vi "UHR-Fleezers Control (host) - Avogadro v2.vi"() -> ()   [LabVIEW 2014] (continued)
              tunnel: w5202 -> [_ w5212]
              frame False {
              }
              frame True {
                n3617 = xnode "Read/Write Control"("FPGA VI Reference In"=w5213, "error in"=w5212, "FPGA Trap Trig"=TRUE) -> ()  [unwired: 2 out]
              }
            }
            n3618 = case shown="True" w5204 {
              frame False {
              }
              frame True {
                w5215 = FALSE ("Value (Signaling)")
                n3619 = local write "Triggered"(w5215) -> ()
                n3620 = local write "Waiting"(TRUE ("Waiting")) -> ()
                n3621 = property on="Green Laser ON" class="Bool (strict)"("Val(Sgnl)"=w5215) -> ()  [unwired: 2 in, 2 out]
              }
            }
          }
          frame "Do nothing" {
          }
          frame "Initialize", Default {
            n3622 = Increment(x=w5226) -> (x+1=w5230:i32)
            n3623 = Select(t=1, s=w5219, f=w5230) -> (s? t:f=w5220:i32)
            n3624 = feedback #23(w5228) -> (w5234:dbl[])
            n3625 = Build Array (concatenate)(w5228, w5234) -> (w5227:dbl[])
            n3626 = Greater Or Equal?(x=w5220, y="Wait to get offset (n)") -> (x >= y?=w5223:bool)
            n3627 = Select(t=w5228, s=w5219, f=w5227) -> (s? t:f=w5229:dbl[])
            n3628 = feedback-in #23(w5229) -> ()
            n3629 = call-poly <vilib>:"Mean.vi"("X"=w5229) -> ("mean"=w5224:dbl)  [unwired: 1 out]
            n3630 = local write "Mean T1 Position\nto compare (nm)"(w5224) -> ()
            n3631 = case shown="True" w5219 {
              tunnel: w5222 -> [_ w5240]
              tunnel: w5221 -> [_ w5239]
              frame False {
              }
              frame True {
                w5236 = FALSE ("FPGA Trap Trig")
                n3632 = xnode "Read/Write Control"("FPGA VI Reference In"=w5240, "error in"=w5239, "FPGA Trap Trig"=w5236) -> ("FPGA VI Reference Out"=w5238:T40, "error out"=w5237:errorcluster)
                n3633 = xnode "Read/Write Control"("FPGA VI Reference In"=w5238, "error in"=w5237, "TTrig?"=w5236) -> ()  [unwired: 2 out]
              }
            }
            n3634 = Select(t="Wait for trigger", s=w5223, f="Initialize") -> (s? t:f=w5231:string)
            n3635 = case shown="True" w5223 {
              tunnel: w5224 -> [_ w5243]
              tunnel: w5222 -> [_ w5252]
              tunnel: w5221 -> [_ w5251]
              frame False {
                n3636 = local write "Waiting"(FALSE ("Waiting")) -> ()
                "Initializing" <- TRUE ("Initializing")
              }
              frame True {
                n3637 = local read "Threshold (nm)"() -> (w5255:dbl)
                n3638 = local read "AOM X Cal (nm/MHz)"() -> (w5254:dbl)
                n3639 = Add(x=w5243, y=w5255) -> (x+y=w5256:dbl)
                n3640 = Divide(x=w5256, y=w5254) -> (x/y=w5253:dbl)
                n3641 = call "IR AOM freq to word.vi"("Frequency In (MHz)"=w5253) -> ("Frequency Word Out (double)"=w5250:dbl)
                n3642 = local write "Initializing"(FALSE ("Initializing")) -> ()
                n3643 = local write "Waiting"(TRUE ("Waiting")) -> ()
                n3644 = To Quad Integer(1:w5250) -> (0:w5249:i64)
                n3645 = xnode "Read/Write Control"("FPGA VI Reference In"=w5252, "error in"=w5251, "FPGA TTrig Thresh"=w5249) -> ("FPGA VI Reference Out"=w5246:T40, "error out"=w5245:errorcluster)
                n3646 = xnode "Read/Write Control"("FPGA VI Reference In"=w5246, "error in"=w5245, "FPGA Trap Trig"=TRUE) -> ()  [unwired: 2 out]
              }
            }
          }
        }
      }
    }
    n3647 = feedback-in #21(w4778) -> ()
    n3648 = feedback-in #22(w4775) -> ()
    n3649 = xnode ("Read/Write Control")("FPGA VI Reference In"=w4570, "error in"=w4837) -> ("FPGA VI Reference Out"=w4567:T40, "error out"=w4763:errorcluster, "AI2 Y Sum Set 1"=w4879:i16, "AI2 Y Sum Set 2"=w4878:i16, "AI1 X Set 1"=w4794:fxp<+/-,16,1>, "AI1 X Set 2"=w4793:fxp<+/-,16,1>, "Trap Pos FB Int Signal"=→"Trap Pos FB Int Signal":fxp<+/-,24,9>, "Trap Pos FB Int-Norm Signal"=→"Trap Pos FB Int-Norm Signal":fxp<+/-,16,1>, "Trap Pos FB Action"=w4787:i64, "Scanning"=→"AOD Scanning":bool, "Scan I"=→"AOD Scan I":u64, "Scanning MCL"=w4881:bool, "Scan I (MCL)"=→"MCL Scan I":u64, "Green FB Sum"=w4844:i16, "Trap Pos FB Action"=w4761:i64, "TTrig Fin Thresh"=w4757:i64, "Red FB Intensity"=w4749:i16, "Blue Intensity"=w4744:i16, "BD1 Frequency Out 1"=w4709:u64)
    "MCL Scanning" <- w4881
    "Trap Pos FB Action" <- w4787
    n3650 = Divide(x=w4749, y=3276.7) -> (x/y=w4748:dbl)
    "Red laser intensity (V)" <- w4748
    n3651 = Divide(x=w4744, y=3276.7) -> (x/y=w4743:dbl)
    "Blue laser intensity (V)" <- w4743
    n3652 = Divide(x=w4844, y=3276.7) -> (x/y=w4747:dbl)
    "Green laser intensity (V)" <- w4747
    n3653 = local read "FB Trig Integrate"() -> (w4755:u32)
    n3654 = Divide(x=w4761, y=w4755) -> (x/y=w4754:dbl)
    "TTrig Sig (Int)" <- w4754
    n3655 = Bundle(w4747, w4748, w4743) -> (→"Fluorescence laser intensities plot":cluster{dbl, dbl, dbl})  [unwired: 1 in]
    n3656 = Divide(x=w4757, y=w4755) -> (x/y=w4752:dbl)
    "TTrig Fin Thresh (Int)" <- w4752
    n3657 = local read "AOM X Cal (nm/MHz)"() -> (w4760:dbl)
    n3658 = local read "AI2 (V)"() -> (w4880:cluster{"Set 1":dbl, "Set 2":dbl})
    n3659 = Bundle By Name(cluster=w4880, "Set 1"=w4879, "Set 2"=w4878) -> (w4711:cluster{"Set 1":dbl, "Set 2":dbl})
    n3660 = Divide(x=w4787, y=327.67) -> (x/y=→"Action (%)":dbl)
    n3661 = case shown="True" "Semi Passive Mode" {
      tunnel: w4617 -> [_ w5028]
      frame False {
      }
      frame True {
        n3662 = local read "Target Force (pN)"() -> (w5026:dbl)
        n3663 = Less?(x="Jump Force (pN)", y=w5026) -> (x < y?=w5024:bool)
        n3664 = case shown="False" w5024 {
          tunnel: "Jump Force (pN)" -> [w5034 w5037]
          tunnel: w5028 -> [w5033 w5036]
          tunnel: [w5032 w5035] -> w5027
          frame False {
            n3665 = Less?(x=w5034, y=w5033) -> (x < y?=w5032:bool)
          }
          frame True {
            n3666 = Greater?(x=w5037, y=w5036) -> (0:w5035:bool)
          }
        }
        n3667 = case shown="False" w5027 {
          frame False {
            n3668 = local read "Trap Pos. FB ON"() -> (w5029:bool)
            n3669 = case shown="False" w5029 {
              frame False {
              }
              frame True {
                n3670 = property on="Trap Pos. FB ON" class="Bool (strict)"("Val(Sgnl)"=FALSE) -> ()  [unwired: 2 in, 2 out]
              }
            }
          }
          frame True {
            n3671 = property on="Trap Pos. FB ON" class="Bool (strict)"("Val(Sgnl)"=TRUE) -> ()  [unwired: 2 in, 2 out]
          }
        }
      }
    }
    n3672 = local read "Trap X (AI1)"() -> (w4807:T19)
    n3673 = call "IR AOM word double to freq.vi"("Frequency Word In (double)"=w4752) -> ("Frequency Out (MHz)"=w4751:dbl)
    n3674 = call "IR AOM word double to freq.vi"("Frequency Word In (double)"=w4754) -> ("Frequency Out (MHz)"=w4753:dbl)
    n3675 = Divide(x=w4711, y=3276.7) -> (x/y=w4876:cluster{"Set 1":dbl, "Set 2":dbl})
    n3676 = Multiply(x=w4753, y=w4760) -> (x*y=w4759:dbl)
    "TTrig Sig (nm)" <- w4759
    n3677 = Multiply(x=w4751, y=w4760) -> (x*y=w4758:dbl)
    "TTrig Fin Thresh (nm)" <- w4758
    n3678 = local write "AI2 (V)"(w4876) -> ()
    n3679 = Bundle(cluster=w4807, "Trap 1"=w4794, "Trap 2"=w4793) -> (→"Trap X (AI1)":T19)
    n3680 = local read "Trap Pos. FB ON"() -> (w4702:bool)
    n3681 = local read "Dynamic Force FB (ronen)"() -> (w4703:bool)
    n3682 = Bundle(w4759, w4758) -> (→"TTrig":cluster{dbl, dbl})  [unwired: 1 in]
    n3683 = Compound Arithmetic op=AND(w4703, "Real time Offset file correction for setpoint", w4702) -> (w4704:bool)
    n3684 = case shown="True" w4704 {
      tunnel: w4709 -> [_ _]
      tunnel: w4640 -> [_ w5056]
      tunnel: w4567 -> [_ w5039]
      frame False {
      }
      frame True {
        # "Changed by Ronen - real time update of set point\naccording to offset file"
        n3685 = local read "T1 calibration"() -> (w5051:T12)
        n3686 = local read "Offset file step size"() -> (w5058:dbl)
        n3687 = local read "Setpoint offset\ncorrection values"() -> (w5055:dbl[])
        n3688 = Multiply(x="Target Force (pN)", y=2.0) -> (x*y=w5052:dbl)
        n3689 = local read "Negate Diff?"() -> (w5040:bool)
        n3690 = Unbundle By Name(w5051) -> ("alpha_x (nm/V)"=w5050:dbl, "kappa_x (pN/nm)"=w5049:dbl)
        n3691 = Divide(x=w5056, y=w5058) -> (x/y=w5059:dbl)
        n3692 = To Long Integer(number=w5059) -> (32bit integer=w5057:i32)
        n3693 = Index Array(array=w5055, index=w5057) -> (element=w5042:dbl)
        n3694 = Multiply(x=w5050, y=w5049) -> (x*y=w5048:dbl)
        n3695 = Select(t=1, s=w5040, f=-1) -> (s? t:f=w5043:i32)
        n3696 = Divide(x=w5052, y=w5048) -> (x/y=w5047:dbl)
        n3697 = Multiply(x=w5043, y=w5042) -> (x*y=w5041:dbl)
        n3698 = Add(x=w5047, y=w5041) -> (x+y=w5046:dbl)
        n3699 = To Fixed-Point(number=w5046) -> (fixed-point=w5038:fxp<+/-,16,1>)  [unwired: 1 in]
        "Actual Setpoint" <- w5038
        n3700 = xnode "Read/Write Control"("FPGA VI Reference In"=w5039, "Trap Pos. FB SP"=w5038) -> ()  [unwired: 1 in, 2 out]
      }
    }
    n3701 = local read "All FB On/Off"() -> (w4710:bool)
    n3702 = case shown="True" w4710 {
      tunnel: w4567 -> [_ w5083]
      frame False {
      }
      frame True {
        n3703 = local read "X RF Amplitude Limits (%)"() -> (w5082:T26)
        n3704 = xnode "Read/Write Control"("FPGA VI Reference In"=w5083) -> ("BD1 amplitude 1 out"=w5074:u16, "BD1 amplitude 2 out"=w5066:u16)  [unwired: 1 in, 2 out]
        n3705 = Unbundle By Name(w5082) -> ("Maximum"=w5065:dbl)
        n3706 = Scale By Power Of 2(n=i16 12, x=ext 1.0) -> (x*2^n=w5078:ext)
        n3707 = Scale By Power Of 2(n=i16 12, x=ext 1.0) -> (x*2^n=w5070:ext)
        n3708 = Subtract(x=w5078, y=ext 1.0) -> (x-y=w5080:ext)
        n3709 = Subtract(x=w5070, y=ext 1.0) -> (x-y=w5068:ext)
        n3710 = Multiply(x=w5074, y=ext 100.0) -> (x*y=w5081:ext)
        n3711 = Multiply(x=w5066, y=ext 100.0) -> (x*y=w5067:ext)
        n3712 = Divide(x=w5081, y=w5080) -> (x/y=w5061:ext)
        "T1 feedback amplitude" <- w5061
        n3713 = Divide(x=w5067, y=w5068) -> (x/y=w5060:ext)
        "T2 feedback amplitude" <- w5060
        n3714 = Greater?(x=w5060, y=w5065) -> (0:w5063:bool)
        n3715 = Greater?(x=w5061, y=w5065) -> (0:w5064:bool)
        n3716 = Or(x=w5064, y=w5063) -> (x .or. y?=w5062:bool)
        n3717 = case shown="True" w5062 {
          frame False {
          }
          frame True {
            n3718 = property on="All FB On/Off" class="Bool (strict)"("Val(Sgnl)"=FALSE) -> ()  [unwired: 2 in, 2 out]
          }
        }
      }
    }
    n3719 = flat-sequence "To save data" {
      tunnel: [w5800] -> w4899
      tunnel: [w5801] -> w4898
      tunnel: w4861 -> [w5794]
      tunnel: w4583 -> [w5798]
      tunnel: ["Save Calibration"] -> w4873
      tunnel: w4692 -> [w5797]
      tunnel: [w5790] -> w4870
      tunnel: [w5787] -> w4869
      tunnel: [w5784] -> w4868
      tunnel: w4860 -> [w5786]
      tunnel: w4648 -> [w5780]
      tunnel: [w5780] -> w4831
      tunnel: ["Start Saving"] -> w4816
      tunnel: [w5775] -> w4783
      tunnel: [w5774] -> w4782
      tunnel: [w5771] -> w4715
      tunnel: [w5767] -> w4708
      tunnel: w4899 -> [w6134]
      tunnel: w4898 -> [w6133]
      tunnel: w4693 -> [w6132]
      tunnel: w4873 -> [w6131]
      tunnel: w4870 -> [w6129]
      tunnel: w4869 -> [w6128]
      tunnel: w4868 -> [w6127]
      tunnel: w4687 -> [w6126]
      tunnel: w4691 -> [w6125]
      tunnel: w4831 -> [w6124]
      tunnel: w4816 -> [w6123]
      tunnel: w4571 -> [w6122]
      tunnel: w4742 -> [w6121]
      tunnel: w4783 -> [w6120]
      tunnel: w4782 -> [w6119]
      tunnel: w4644 -> [w6118]
      tunnel: w4653 -> [w6117]
      tunnel: w4690 -> [w6116]
      tunnel: w4715 -> [w6115]
      tunnel: w4708 -> [w6114]
      frame #0 {
        # "Changed by Ronen - we don't have a database so we disabled this"
        n3720 = Or(x="Save N Sets", y="Start Saving") -> (x .or. y?=w5781:bool)
        n3721 = To Double Precision Float(number=w5797) -> (double precision float=w5791:dbl)
        n3722 = Build Array(w5781, "Save Calibration", w5794, w5786, "Flow Cal") -> (w5796:bool[])
        n3723 = Compound Arithmetic op=OR("Save Calibration", w5794, w5781, w5786, "Flow Cal") -> (w5799:bool)
        n3724 = Boolean Array To Number(Boolean array=w5796) -> (number=w5793:u32)
        n3725 = feedback #24(FALSE ("Save APD Data\nwith Trap Data")) -> (w5776:bool)
        n3726 = feedback #25(refnum<k0> refnum) -> (w5802:refnum<file>)
        n3727 = feedback #26(FALSE ("Save APD Data\nwith Trap Data")) -> (w5785:bool)
        n3728 = feedback #27(0) -> (w5804:i32)
        n3729 = feedback #28() -> (w5792:u32)  [unwired: 1 out]
        n3730 = feedback #29(refnum<k0> refnum) -> (w5772:refnum<file>)
        n3731 = feedback #30(refnum<k0> refnum) -> (w5778:refnum<file>)
        n3732 = feedback #31(refnum<k0> refnum) -> (w5768:refnum<file>)
        n3733 = feedback #32(refnum<k0> refnum) -> (w5788:refnum<file>)
        n3734 = case shown="True" w5799 {
          tunnel: [w5813 1] -> w5800
          tunnel: w5804 -> [w5815 _]
          tunnel: [w5814 w5847] -> w5801
          tunnel: w5802 -> [w5814 _]
          tunnel: w5798 -> [_ w5865]
          tunnel: w5791 -> [_ w5863]
          tunnel: w5793 -> [_ w5866]
          tunnel: [w5812 w5846] -> w5790
          tunnel: w5792 -> [w5812 _]
          tunnel: [w5811 w5844] -> w5787
          tunnel: w5788 -> [w5811 _]
          tunnel: [w5810 w5843] -> w5784
          tunnel: w5785 -> [w5810 _]
          tunnel: "Start Saving" -> [_ w5841]
          tunnel: w5780 -> [_ w5840]
          tunnel: [w5809 w5833] -> w5774
          tunnel: w5778 -> [w5809 _]
          tunnel: [w5808 w5832] -> w5775
          tunnel: w5776 -> [w5808 _]
          tunnel: [w5807 w5818] -> w5771
          tunnel: w5772 -> [w5807 _]
          tunnel: [w5806 w5816] -> w5767
          tunnel: w5768 -> [w5806 _]
          frame False {
            n3735 = Increment(x=w5815) -> (x+1=w5813:i32)
          }
          frame True {
            w5817 = FALSE ("Start Saving")
            w5842 = 10.0  # File Version
            w5849 = FALSE ("prepend array or string size? (T)")
            w5848 = T53."big-endian, network order" ("byte order (0:big-endian, network order)")
            # "RG added position values of traps in the saved\nfile for AOD rasters and time series."
            # "Ronen Changed the create file - changed data folder to c:\\Data"
            # "Save trap position\ndata"
            n3736 = Array Size(array=w5840) -> (size(s)=w5839:i32)
            n3737 = To Double Precision Float(number=w5839) -> (double precision float=w5838:dbl)
            n3738 = local read "BD 1 Frequency 1 (MHz)"() -> (w5862:dbl)
            n3739 = local read "BD 2 Frequency 1 (MHz)"() -> (w5861:dbl)
            n3740 = local read "BD 1 Frequency 2 (MHz)"() -> (w5860:dbl)
            n3741 = local read "BD 2 Frequency 2 (MHz)"() -> (w5859:dbl)
            n3742 = local read "BD 1 Frequency 3 (MHz)"() -> (w5858:dbl)
            n3743 = local read "BD 2 Frequency 3 (MHz)"() -> (w5857:dbl)
            n3744 = local write "Flow Cal"(w5817) -> ()
            n3745 = local write "Save Calibration"(w5817) -> ()
            n3746 = local write "Start Saving"(w5817) -> ()
            n3747 = Build Array("Save APD Data\nwith Trap Data", "Save Trap Pos. Data") -> (w5835:bool[])
            n3748 = Boolean Array To Number(Boolean array=w5835) -> (number=w5834:u32)
            n3749 = Build Array(w5862, w5861, w5860, w5859, w5858, w5857) -> (w5856:dbl[])
            n3750 = case shown="1, Default" w5866 {
              tunnel: w5865 -> [w5972 w5999 w6031 w6069 w6106]
              tunnel: w5838 -> [w5977 w6006 w6051 w6088 w6111]
              tunnel: w5863 -> [w5976 w6005 w6050 w6087 w6110]
              tunnel: [w5973 w6001 w6042 w6079 w6107] -> w5854
              tunnel: [w5964 "Cal sets to save" w6032 w6070 w6093] -> w5846
              tunnel: w5856 -> [w5974 w6002 w6044 w6081 w6108]
              tunnel: "Save APD Data\nwith Trap Data" -> [w5971 w5988 w6029 w6067 w6105]
              tunnel: [w5971 w5986 w6029 w6067 w6105] -> w5843
              tunnel: w5842 -> [w5967 w5995 w6027 w6065 w6101]
              tunnel: w5841 -> [w5966 _ _ _ _]
              tunnel: [w5957 w5994 w6026 w6055 w6100] -> w5832
              tunnel: "Save Trap Pos. Data" -> [w5957 w5993 w6026 w6055 w6100]
              tunnel: w5834 -> [w5956 w5992 w6025 w6054 w6099]
              frame 1, Default {
                # "timeseries"
                n3751 = case shown="True" "Profile" {
                  tunnel: [w5980 w5984] -> w5961
                  tunnel: [w5980 w5983] -> w5960
                  tunnel: [w5980 w5982] -> w5959
                  tunnel: [w5980 w5981] -> w5958
                  frame False {
                    w5980 = 0.0 ("f")
                  }
                  frame True {
                    n3752 = local read "Current Position"() -> (w5985:cluster{dbl, dbl, dbl})
                    n3753 = local read "Y change (mm)"() -> (w5981:dbl)
                    n3754 = Unbundle(w5985) -> (w5984:dbl, w5983:dbl, w5982:dbl)
                  }
                }
                n3755 = local read "Save ave N"() -> (w5979:dbl)
                n3756 = local read "AOM X Cal (nm/MHz)"() -> (w5955:dbl)
                n3757 = local read "Piezo Trap X cal (nm/V)"() -> (w5954:dbl)
                n3758 = local read "Piezo Trap Y cal (nm/V)"() -> (w5953:dbl)
                n3759 = local read "Piezo trap x\noffset (V)"() -> (w5952:dbl)
                n3760 = local read "Piezo trap y\noffset (V)"() -> (w5951:dbl)
                n3761 = To Double Precision Float(number=w5956) -> (double precision float=w5970:dbl)
                n3762 = Multiply(x=w5979, y=w5972) -> (x*y=w5978:dbl)
                n3763 = Build Array(w5967, w5972, w5978, w5977, w5976, 0.0 ("f")) -> (w5975:dbl[])
                n3764 = Build Array(w5970, w5961, w5960, w5959, w5958) -> (w5968:dbl[])
                n3765 = Build Array(w5955, w5954, w5953, w5952, w5951) -> (w5950:dbl[])
                n3766 = Select(t=u32 4000000000, s=w5966, f="N sets to save") -> (s? t:f=w5964:u32)
                n3767 = Build Array (concatenate)(w5975, w5974, w5968, w5950) -> (w5973:dbl[])
              }
              frame 2 {
                w5997 = 0.0 ("f")
                w5987 = FALSE ("Save APD Data\nwith Trap Data")
                # "For diagnostics save trap position\ndata during cal"
                # "calibration"
                n3768 = Boolean To (0,1)(Boolean=w5987) -> (0, 1=w5991:i16)
                n3769 = Select(t=w5988, s="Save trap pos with cal", f=w5987) -> (s? t:f=w5986:bool)
                n3770 = Select(t=w5993, s="Save trap pos with cal", f=w5987) -> (s? t:f=w5994:bool)
                n3771 = Select(t=w5992, s="Save trap pos with cal", f=w5991) -> (s? t:f=w5990:u32)
                n3772 = To Double Precision Float(number=w5990) -> (double precision float=w5998:dbl)
                n3773 = Build Array(w5995, w5999, w5999, w6006, w6005, 1.0 ("t")) -> (w6003:dbl[])
                n3774 = Build Array(w5998, w5997, w5997, w5997, w5997) -> (w5996:dbl[])
                n3775 = Build Array (concatenate)(w6003, w6002, w5996) -> (w6001:dbl[])
                "Calibrating Trap..." <- TRUE ("Calibrating...")
              }
              frame 4 {
                # "scan dir (x/y = 0/1)"
                # "cycles/step"
                # "n scans (f/b)"
                # "steps"
                # "freq. range"
                # "AOD raster scan"
                n3776 = local read "MCL offset scanning range (V)"() -> (w6022:T4)
                n3777 = local read "Multiple-MCL offset?"() -> (w6017:bool)
                n3778 = local read "Piezo Trap Y cal (nm/V)"() -> (w6008:dbl)
                n3779 = local read "AOM X Cal (nm/MHz)"() -> (w6010:dbl)
                n3780 = local read "Piezo Trap X cal (nm/V)"() -> (w6011:dbl)
                n3781 = local read "Piezo trap x\noffset (V)"() -> (w6012:dbl)
                n3782 = local read "Piezo trap y\noffset (V)"() -> (w6013:dbl)
                n3783 = local read "Number of F/B Scans (AOD)"() -> (w6036:u16)
                n3784 = Boolean To (0,1)(Boolean="Offset raster?") -> (0, 1=w6015:i16)
                n3785 = call "Make Trap3 position array.vi"("MCL offset scanning range (V)"=w6022) -> ("X Data points"=w6021:u64, "Y data points"=w6020:u64)  [unwired: 3 out]
                n3786 = Boolean To (0,1)(Boolean=w6017) -> (0, 1=w6024:i16)
                n3787 = local read "Cycles/step (AOD)"() -> (w6038:u64)
                n3788 = local read "Scan Range (MHz)"() -> (w6041:dbl)
                n3789 = local read "Scan steps (AOD)"() -> (w6040:u64)
                n3790 = local read "Scan BD"() -> (w6048:bool)
                n3791 = To Double Precision Float(number=w6024) -> (double precision float=w6023:dbl)
                n3792 = local read "Save ave N"() -> (w6053:dbl)
                n3793 = To Double Precision Float(number=w6020) -> (double precision float=w6018:dbl)
                n3794 = Build Array(w6010, w6011, w6008, w6012, w6013) -> (w6009:dbl[])
                n3795 = To Double Precision Float(number=w6021) -> (double precision float=w6019:dbl)
                n3796 = Boolean To (0,1)(Boolean=w6048) -> (0, 1=w6047:i16)
                n3797 = To Double Precision Float(number=w6015) -> (double precision float=w6014:dbl)
                n3798 = To Double Precision Float(number=w6036) -> (double precision float=w6035:dbl)
                n3799 = To Double Precision Float(number=w6040) -> (double precision float=w6039:dbl)
                n3800 = To Double Precision Float(number=w6038) -> (double precision float=w6037:dbl)
                n3801 = To Double Precision Float(number=w6047) -> (double precision float=w6046:dbl)
                n3802 = Multiply(x=w6053, y=w6031) -> (x*y=w6052:dbl)
                n3803 = To Double Precision Float(number=w6025) -> (double precision float=w6030:dbl)
                n3804 = local read "N sets should be saved"() -> (w6033:dbl)
                n3805 = Build Array(w6030, w6023, w6019, w6018, w6014) -> (w6028:dbl[])
                n3806 = Build Array(w6046, w6041, w6039, w6037, w6035) -> (w6043:dbl[])
                n3807 = Build Array(w6027, w6031, w6052, w6051, w6050, 2.0 ("t")) -> (w6045:dbl[])
                n3808 = Build Array (concatenate)(w6045, w6044, w6028, w6043, w6009) -> (w6042:dbl[])
                n3809 = Round Toward +Infinity(x=w6033) -> (ceil(x): smallest int >= x=w6034:dbl)
                n3810 = To Unsigned Long Integer(number=w6034) -> (unsigned 32bit integer=w6032:u32)
              }
              frame 8 {
                w6062 = 0.0 ("f")
                # "MCL raster scan"
                n3811 = local read "Number of scans (MCL)"() -> (w6057:u64)
                n3812 = local read "2D or 1D Scan"() -> (w6059:bool)
                n3813 = local read "Scan lines (y)"() -> (w6056:u64)
                n3814 = local read "Scan Range (V)\n(of steps)"() -> (w6078:dbl)
                n3815 = local read "Fast Scan Dir"() -> (w6085:bool)
                n3816 = local read "Cycles/step (MCL)"() -> (w6075:u64)
                n3817 = local read "Scan steps (MCL)"() -> (w6077:u64)
                n3818 = Select(t=w6056, s=w6059, f=w6057) -> (s? t:f=w6058:u64)
                n3819 = Boolean To (0,1)(Boolean=w6059) -> (0, 1=w6061:i16)
                n3820 = local read "Save ave N"() -> (w6090:dbl)
                n3821 = local read "Initial X"() -> (w6064:dbl)
                n3822 = local read "Initial Y"() -> (w6063:dbl)
                n3823 = To Double Precision Float(number=w6061) -> (double precision float=w6060:dbl)
                n3824 = Boolean To (0,1)(Boolean=w6085) -> (0, 1=w6084:i16)
                n3825 = To Double Precision Float(number=w6058) -> (double precision float=w6073:dbl)
                n3826 = To Double Precision Float(number=w6077) -> (double precision float=w6076:dbl)
                n3827 = To Double Precision Float(number=w6075) -> (double precision float=w6074:dbl)
                n3828 = To Double Precision Float(number=w6084) -> (double precision float=w6083:dbl)
                n3829 = Multiply(x=w6090, y=w6069) -> (x*y=w6089:dbl)
                n3830 = To Double Precision Float(number=w6054) -> (double precision float=w6068:dbl)
                n3831 = local read "N sets should be saved (MCL)"() -> (w6071:dbl)
                n3832 = Build Array(w6068, w6060, w6062, w6062, w6062) -> (w6066:dbl[])
                n3833 = Build Array(w6083, w6078, w6076, w6074, w6073, w6064, w6063) -> (w6080:dbl[])
                n3834 = Build Array(w6065, w6069, w6089, w6088, w6087, 3.0 ("t")) -> (w6082:dbl[])
                n3835 = Round Toward +Infinity(x=w6071) -> (ceil(x): smallest int >= x=w6072:dbl)
                n3836 = Build Array (concatenate)(w6082, w6081, w6066, w6080) -> (w6079:dbl[])
                n3837 = To Unsigned Long Integer(number=w6072) -> (unsigned 32bit integer=w6070:u32)
              }
              frame 16 {
                w6092 = 0.0
                # "Flow calibration - added by Ronen: Number\nof saved sets is distance (1 mm) divided by \nspeed +1.5 spare second divided by the time of\nset measurement, 0.2 sec for 2 set interlace"
                # "timeseries"
                n3838 = local read "Save ave N"() -> (w6113:dbl)
                n3839 = Reciprocal(x=0.0) -> (1/x=w6098:dbl)
                n3840 = Add(x=w6098, y=1.5) -> (x+y=w6096:dbl)
                n3841 = Multiply(x=w6113, y=w6106) -> (x*y=w6112:dbl)
                n3842 = Divide(x=w6096, y=0.2) -> (x/y=w6094:dbl)
                n3843 = To Double Precision Float(number=w6099) -> (double precision float=w6104:dbl)
                n3844 = To Unsigned Long Integer(number=w6094) -> (unsigned 32bit integer=w6093:u32)
                n3845 = Build Array(w6101, w6106, w6112, w6111, w6110, 4.0 ("f")) -> (w6109:dbl[])
                n3846 = Build Array(w6104, w6092, w6092, w6092, w6092) -> (w6102:dbl[])
                n3847 = Build Array (concatenate)(w6109, w6108, w6102) -> (w6107:dbl[])
              }
            }
            n3848 = local read "Index"() -> (w5871:dbl)
            n3849 = call "Create new save file.vi"("Insert"="", "Ext"=".dat", "Index In"=w5871) -> ("Path Out"=w5820:path, "Index Out"=w5845:dbl)
            n3850 = local write "Save file name"(w5820) -> ()
            n3851 = local write "Index"(w5845) -> ()
            n3852 = local write "Save index"(w5845) -> ()
            n3853 = case shown="True" "Save Event Log?" {
              tunnel: w5820 -> [_ w5885]
              tunnel: [refnum<k0> refnum w5884] -> w5818
              frame False {
              }
              frame True {
                (unwired) FALSE ("prepend array or string size? (T)")
                n3854 = Path To String(path=w5885) -> (string=w5896:string)
                n3855 = String Length(string=w5896) -> (length=w5895:i32)
                n3856 = Subtract(x=w5895, y=4) -> (x-y=w5893:i32)
                n3857 = String Subset(string=w5896, length (rest)=w5893) -> (substring=w5892:string)  [unwired: 1 out]
                n3858 = Concatenate Strings(w5892, "_log.txt" ("string")) -> (w5890:string)
                n3859 = String To Path(string=w5890) -> (path=w5886:path)
                n3860 = Open/Create/Replace File(file path (use dialog)=w5886, operation (0:open)=T52."create", access (0:read/write)=enum16{"read/write", "read-only", "write-only"}."write-only") -> (refnum out=w5887:refnum<file>)  [unwired: 1 in, 4 out]
                n3861 = Deny Access(7:w5887) -> (3:w5884:refnum<file>)  [unwired: 1 in, 2 out]
                n3862 = call "write to event log.vi"("log file ref"=w5884, "time"=0.0, "input string"="start log") -> ()  [unwired: 8 in]
              }
            }
            "log file ref" <- w5818
            n3863 = Array Size(array=w5854) -> (size(s)=w5855:i32)
            n3864 = Open/Create/Replace File(file path (use dialog)=w5820, operation (0:open)=T52."create", access (0:read/write)=enum16{"read/write", "read-only", "write-only"}."write-only") -> (refnum out=w5868:refnum<file>)  [unwired: 1 in, 4 out]
            n3865 = local write "Saving..."(TRUE ("Saving...")) -> ()
            n3866 = To Double Precision Float(number=w5855) -> (double precision float=w5853:dbl)
            n3867 = String Length(string="Comment (data description)") -> (length=w5852:i32)
            n3868 = To Double Precision Float(number=w5852) -> (double precision float=w5851:dbl)
            n3869 = Deny Access(7:w5868) -> (3:w5867:refnum<file>)  [unwired: 1 in, 2 out]
            n3870 = Build Array (concatenate)(w5853, w5854, w5851) -> (w5830:dbl[])
            n3871 = case "If fluorescence data to be saved" shown="True" w5843 {
              tunnel: w5820 -> [_ w5949]
              tunnel: [w5919 w5932] -> w5844
              tunnel: [w5919 w5920] -> w5816
              frame False {
                w5919 = refnum<k0> refnum
              }
              frame True {
                w5931 = 0.0
                w5924 = T52."create" ("operation (0:open)")
                w5925 = enum16{"read/write", "read-only", "write-only"}."write-only" ("access (0:read/write)")
                n3872 = local read "APD Integration Time (s)"() -> (w5937:dbl)
                n3873 = local read "N APD Samp/step"() -> (w5930:dbl)
                n3874 = local read "Number of APDs"() -> (w5929:u8)
                n3875 = Path To String(path=w5949) -> (string=w5948:string)
                n3876 = String Length(string=w5948) -> (length=w5947:i32)
                n3877 = Subtract(x=w5947, y=4) -> (x-y=w5945:i32)
                n3878 = String Subset(string=w5948, length (rest)=w5945) -> (substring=w5928:string)  [unwired: 1 out]
                n3879 = Build Array(w5937, w5930, w5929, w5931, w5931, w5931, w5931, w5931) -> (w5934:dbl[])
                n3880 = Concatenate Strings(w5928, "_green.dat") -> (w5926:string)
                n3881 = Concatenate Strings(w5928, "_fl.dat" ("string")) -> (w5943:string)
                n3882 = Array Size(array=w5934) -> (size(s)=w5936:i32)
                n3883 = String To Path(string=w5943) -> (path=w5941:path)
                n3884 = Open/Create/Replace File(file path (use dialog)=w5941, operation (0:open)=w5924, access (0:read/write)=w5925) -> (refnum out=w5942:refnum<file>)  [unwired: 1 in, 4 out]
                n3885 = Deny Access(7:w5942) -> (3:w5938:refnum<file>)  [unwired: 1 in, 2 out]
                n3886 = String To Path(string=w5926) -> (path=w5923:path)
                n3887 = To Double Precision Float(number=w5936) -> (double precision float=w5935:dbl)
                n3888 = Build Array (concatenate)(w5935, w5934) -> (w5933:dbl[])
                n3889 = Write to Binary File(file (use dialog)=w5938, data=w5933, 5:FALSE ("prepend array or string size? (T)"), 9:T53."big-endian, network order" ("byte order (0:big-endian, network order)")) -> (refnum out=w5932:refnum<file>)  [unwired: 1 in, 3 out]
                n3890 = Open/Create/Replace File(file path (use dialog)=w5923, operation (0:open)=w5924, access (0:read/write)=w5925) -> (refnum out=w5921:refnum<file>, error out=w5922:errorcluster)  [unwired: 3 in, 1 out]
                n3891 = Deny Access(4:w5922, 7:w5921) -> (3:w5920:refnum<file>)  [unwired: 1 in, 1 out]
              }
            }
            n3892 = case shown="True" w5832 {
              tunnel: w5820 -> [_ w5904]
              tunnel: [refnum<k0> refnum w5903] -> w5833
              frame False {
              }
              frame True {
                w5899 = 0.0 ("element")
                n3893 = Path To String(path=w5904) -> (string=w5918:string)
                n3894 = Build Array(w5899, w5899, w5899, w5899, w5899, w5899, w5899, w5899) -> (w5900:dbl[])
                n3895 = String Length(string=w5918) -> (length=w5917:i32)
                n3896 = Subtract(x=w5917, y=4) -> (x-y=w5915:i32)
                n3897 = Array Size(array=w5900) -> (size(s)=w5902:i32)
                n3898 = String Subset(string=w5918, length (rest)=w5915) -> (substring=w5914:string)  [unwired: 1 out]
                n3899 = To Double Precision Float(number=w5902) -> (double precision float=w5901:dbl)
                n3900 = Concatenate Strings(w5914, "_pos.dat" ("string")) -> (w5912:string)
                n3901 = Build Array (concatenate)(w5901, w5900) -> (w5898:dbl[])
                n3902 = String To Path(string=w5912) -> (path=w5908:path)
                n3903 = Open/Create/Replace File(file path (use dialog)=w5908, operation (0:open)=T52."create", access (0:read/write)=enum16{"read/write", "read-only", "write-only"}."write-only") -> (refnum out=w5909:refnum<file>)  [unwired: 1 in, 4 out]
                n3904 = Deny Access(7:w5909) -> (3:w5905:refnum<file>)  [unwired: 1 in, 2 out]
                n3905 = Write to Binary File(file (use dialog)=w5905, data=w5898, 5:FALSE ("prepend array or string size? (T)"), 9:T53."big-endian, network order" ("byte order (0:big-endian, network order)")) -> (refnum out=w5903:refnum<file>)  [unwired: 1 in, 3 out]
              }
            }
            n3906 = Write to Binary File(file (use dialog)=w5867, data=w5830, 5:w5849, 9:w5848) -> (refnum out=w5850:refnum<file>)  [unwired: 1 in, 3 out]
            n3907 = Write to Binary File(file (use dialog)=w5850, data="Comment (data description)", 5:w5849, 9:w5848) -> (refnum out=w5847:refnum<file>)  [unwired: 1 in, 3 out]
            n3908 = local read "connection reference"() -> (w5831:T27)
            n3909 = Bundle("Comment (data description)"="Comment (data description)", "Channel 1 Buffer"="Channel 1 Buffer", "Channel 2 Buffer"="Channel 2 Buffer", "Channel 3 Buffer"="Channel 3 Buffer", "Title"="Title", "DNA Construct"="DNA Construct", "Bead diameter"="Bead diameter", "Name"="Name") -> (w5821:T74)  [unwired: 1 in]
            n3910 = disable-structure shown="Disabled" {
              disable-tunnel: w5831 -> [w5879 _]
              disable-tunnel: w5830 -> [w5877 _]
              disable-tunnel: w5821 -> [w5876 _]
              disable-tunnel: w5820 -> [w5875 _]
              frame Disabled {
                n3911 = call "MattFileCreator-v9.vi"("Comments"=w5876, "Input Array"=w5877, "File path"=w5875, "table"="labview", "connection reference"=w5879) -> ("connection reference out"=w5878:T27)  [unwired: 5 in, 1 out]
                n3912 = local write "connection reference"(w5878) -> ()
              }
              frame Enabled {
              }
            }
          }
        }
        n3913 = feedback-in #24(w5775) -> ()
        n3914 = feedback-in #25(w5801) -> ()
        n3915 = feedback-in #26(w5784) -> ()
        n3916 = feedback-in #27(w5800) -> ()
        n3917 = feedback-in #28(w5790) -> ()
        n3918 = feedback-in #29(w5771) -> ()
        n3919 = feedback-in #30(w5774) -> ()
        n3920 = feedback-in #31(w5767) -> ()
        n3921 = feedback-in #32(w5787) -> ()
      }
      frame #1 {
        n3922 = local read "Saving..."() -> (w6130:bool)
        n3923 = case shown="True" w6130 {
          tunnel: w6134 -> [_ w6148]
          tunnel: w6133 -> [_ w6162]
          tunnel: w6132 -> [_ w6158]
          tunnel: w6131 -> [_ w6157]
          tunnel: w6129 -> [_ w6156]
          tunnel: w6128 -> [_ w6151]
          tunnel: w6127 -> [_ w6150]
          tunnel: w6126 -> [_ w6149]
          tunnel: w6125 -> [_ w6147]
          tunnel: w6124 -> [_ w6145]
          tunnel: w6123 -> [_ w6144]
          tunnel: w6122 -> [_ w6143]
          tunnel: w6121 -> [_ w6142]
          tunnel: w6120 -> [_ w6141]
          tunnel: w6119 -> [_ w6140]
          tunnel: w6118 -> [_ w6139]
          tunnel: w6117 -> [_ w6138]
          tunnel: w6116 -> [_ w6137]
          tunnel: w6115 -> [_ w6136]
          tunnel: w6114 -> [_ w6135]
          frame False {
          }
          frame True {
            n3924 = Multiply(x=w6148, y=w6147) -> (x*y=→"Time (s)":dbl)
            n3925 = Less Or Equal?(x=w6148, y=w6156) -> (x <= y?=w6160:bool)
            n3926 = Compound Arithmetic op=OR("Stop Saving", "Abort save 2") -> (w6152:bool)
            n3927 = Not(x=w6152) -> (.not. x?=w6161:bool)
            n3928 = And(x=w6160, y=w6161) -> (x .and. y?=w6159:bool)
            n3929 = case shown="True" w6159 {
              tunnel: w6162 -> [w6172 w6273]
              tunnel: [0.0 w6276] -> w6155
              tunnel: w6148 -> [_ w6274]
              tunnel: w6156 -> [_ w6275]
              tunnel: w6158 -> [_ w6270]
              tunnel: w6157 -> [_ _]
              tunnel: w6151 -> [w6170 w6263]
              tunnel: w6150 -> [w6169 w6264]
              tunnel: w6149 -> [_ w6262]
              tunnel: w6145 -> [_ w6261]
              tunnel: w6144 -> [_ w6179]
              tunnel: w6143 -> [_ w6254]
              tunnel: w6142 -> [_ w6201]
              tunnel: w6141 -> [w6166 w6218]
              tunnel: w6140 -> [w6167 w6217]
              tunnel: w6139 -> [_ w6214]
              tunnel: w6138 -> [_ w6212]
              tunnel: w6137 -> [_ w6178]
              tunnel: w6136 -> [w6165 _]
              tunnel: w6135 -> [w6163 w6177]
              frame False {
                w6168 = FALSE
                n3930 = Close File(refnum=w6172) -> ()  [unwired: 1 in, 2 out]
                n3931 = case shown="True" w6169 {
                  tunnel: w6170 -> [_ w6176]
                  tunnel: w6163 -> [_ w6175]
                  frame False {
                  }
                  frame True {
                    n3932 = Close File(refnum=w6176) -> ()  [unwired: 1 in, 2 out]
                    n3933 = Close File(refnum=w6175) -> ()  [unwired: 1 in, 2 out]
                  }
                }
                n3934 = case shown="True" w6166 {
                  tunnel: w6167 -> [_ w6174]
                  frame False {
                  }
                  frame True {
                    n3935 = Close File(refnum=w6174) -> ()  [unwired: 1 in, 2 out]
                  }
                }
                n3936 = local read "Save Event Log?"() -> (w6164:bool)
                n3937 = case shown="True" w6164 {
                  tunnel: w6165 -> [_ w6173]
                  frame False {
                  }
                  frame True {
                    n3938 = Close File(refnum=w6173) -> ()  [unwired: 1 in, 2 out]
                  }
                }
                n3939 = local write "Raster Scanning..."(w6168) -> ()
                n3940 = local write "Calibrating Trap..."(w6168) -> ()
                n3941 = call <vilib>:"Beep.vi"() -> ()  [unwired: 3 in, 9 out]
                n3942 = local write "Stop Saving"(w6168) -> ()
                "Saving..." <- w6168
              }
              frame True {
                n3943 = local read "Calibrating Trap..."() -> (w6265:bool)
                n3944 = case "Write fl. data" shown="True" w6264 {
                  tunnel: w6263 -> [_ w6306]
                  tunnel: w6262 -> [_ w6305]
                  tunnel: w6177 -> [_ w6299]
                  frame False {
                  }
                  frame True {
                    w6298 = FALSE ("prepend array or string size? (T)")
                    w6300 = T53."big-endian, network order" ("byte order (0:big-endian, network order)")
                    n3945 = property on="Green Laser ON" class="Bool (strict)"() -> ("Value"=w6304:bool)  [unwired: 2 in, 2 out]
                    n3946 = property on="Green Intensity % (FB OFF)" class="DigNum (strict)"() -> ("Value"=w6303:dbl)  [unwired: 2 in, 2 out]
                    n3947 = Boolean To (0,1)(Boolean=w6304) -> (0, 1=w6302:i16)
                    n3948 = Multiply(x=w6302, y=w6303) -> (x*y=w6301:dbl)
                    n3949 = Write to Binary File(file (use dialog)=w6306, data=w6305, 5:w6298, 9:w6300) -> ()  [unwired: 1 in, 4 out]
                    n3950 = Write to Binary File(file (use dialog)=w6299, data=w6301, 5:w6298, 9:w6300) -> ()  [unwired: 2 in, 3 out]
                  }
                }
                n3951 = Greater?(x="Save ave N", y=1.0) -> (0:w6268:bool)
                n3952 = Not(x=w6265) -> (.not. x?=w6267:bool)
                n3953 = And(x=w6267, y=w6268) -> (x .and. y?=w6215:bool)
                n3954 = case shown="True" w6215 {
                  tunnel: w6214 -> [w6279 w6290]
                  tunnel: [w6279 w6282] -> w6213
                  tunnel: "Save ave N" -> [_ w6283]
                  frame False {
                  }
                  frame True {
                    w6280 = 4 ("dimension size")
                    n3955 = Array Size(array=w6290) -> (size(s)=w6284:i32)
                    n3956 = Divide(x=w6284, y=w6280) -> (x/y=w6288:dbl)
                    n3957 = Reshape Array(w6290, w6288, w6280) -> (w6289:u64[][])
                    n3958 = Transpose 2D Array(2D array=w6289) -> (transposed array=w6287:u64[][])
                    n3959 = for {
                      tunnel: w6287 -> [w6292] mode=indexing
                      tunnel: [w6291] -> w6281 mode=indexing
                      tunnel: w6283 -> [w6293]
                      workers-P: _ -> [_]
                      n3960 = call "downsample 1D array - U64.vi"("Ave N"=w6293, "Array In"=w6292) -> ("Array Out"=w6291:u64[])  [unwired: 1 in]
                    }
                    n3961 = Transpose 2D Array(2D array=w6281) -> (transposed array=w6286:u64[][])
                    n3962 = Divide(x=w6284, y=w6283) -> (x/y=w6285:dbl)
                    n3963 = Reshape Array(w6286, w6285) -> (w6282:u64[])
                  }
                }
                n3964 = case shown="True" w6215 {
                  tunnel: w6270 -> [w6307 w6319]
                  tunnel: [w6307 w6311] -> w6266
                  tunnel: "Save ave N" -> [_ w6312]
                  tunnel: w6261 -> [_ w6310]
                  frame False {
                  }
                  frame True {
                    n3965 = Array Size(array=w6319) -> (size(s)=w6313:i32)
                    n3966 = Array Size(array=w6310) -> (size(s)=w6309:i32)
                    n3967 = Divide(x=w6313, y=w6309) -> (x/y=w6317:dbl)
                    n3968 = Reshape Array(w6319, w6317, w6309) -> (w6318:i16[][])
                    n3969 = Transpose 2D Array(2D array=w6318) -> (transposed array=w6316:i16[][])
                    n3970 = for {
                      tunnel: w6316 -> [w6322] mode=indexing
                      tunnel: [w6321] -> w6308 mode=indexing
                      tunnel: w6312 -> [w6320]
                      workers-P: _ -> [_]
                      n3971 = call "downsample 1D array - I16 to F32.vi"("Ave N"=w6320, "Array In"=w6322) -> ("Array Out"=w6321:sgl[])  [unwired: 1 in]
                    }
                    n3972 = Transpose 2D Array(2D array=w6308) -> (transposed array=w6315:sgl[][])
                    n3973 = Divide(x=w6313, y=w6312) -> (x/y=w6314:dbl)
                    n3974 = Reshape Array(w6315, w6314) -> (w6311:sgl[])
                  }
                }
                n3975 = Index Array(array=w6201, index=2) -> (element=w6202:waveform(dbl))
                n3976 = Index Array(array=w6201, index=1) -> (element=w6235:waveform(dbl))
                n3977 = Index Array(array=w6201, index=0) -> (element=w6237:waveform(dbl))
                n3978 = Unbundle By Name(w6202) -> ("Y"=w6204:dbl[])
                n3979 = Unbundle By Name(w6235) -> ("Y"=w6239:dbl[])
                n3980 = Unbundle By Name(w6237) -> ("Y"=w6247:dbl[])
                n3981 = case "Write trap pos. data" shown="True" w6218 {
                  tunnel: w6217 -> [_ w6295]
                  tunnel: w6213 -> [_ w6294]
                  frame False {
                  }
                  frame True {
                    n3982 = Write to Binary File(file (use dialog)=w6295, data=w6294, 5:FALSE ("prepend array or string size? (T)"), 9:T53."big-endian, network order" ("byte order (0:big-endian, network order)")) -> ()  [unwired: 1 in, 4 out]
                  }
                }
                n3983 = Write to Binary File(file (use dialog)=w6273, data=w6266, 5:FALSE ("prepend array or string size? (T)"), 9:T53."big-endian, network order" ("byte order (0:big-endian, network order)")) -> ()  [unwired: 1 in, 4 out]
                n3984 = feedback #33(w6204) -> (w6205:dbl[])
                n3985 = Build Array (concatenate)(w6205, w6204) -> (w6200:dbl[])
                n3986 = Select(t=w6204, s=w6179, f=w6200) -> (s? t:f=w6190:dbl[])
                n3987 = feedback-in #33(w6190) -> ()
                n3988 = feedback #34(w6239) -> (w6241:dbl[])
                n3989 = Build Array (concatenate)(w6241, w6239) -> (w6240:dbl[])
                n3990 = Select(t=w6239, s=w6179, f=w6240) -> (s? t:f=w6229:dbl[])
                n3991 = feedback-in #34(w6229) -> ()
                n3992 = feedback #35(w6247) -> (w6260:dbl[])
                n3993 = Build Array (concatenate)(w6260, w6247) -> (w6259:dbl[])
                n3994 = Select(t=w6247, s=w6179, f=w6259) -> (s? t:f=w6234:dbl[])
                n3995 = feedback-in #35(w6234) -> ()
                n3996 = Divide(x=w6274, y=w6275) -> (x/y=w6277:dbl)
                n3997 = Multiply(x=w6277, y=100.0) -> (x*y=w6276:dbl)
                n3998 = Build Array(w6234, w6229, w6190) -> (→"Saved APD":dbl[][])
                n3999 = Array Size(array=w6234) -> (size(s)=w6252:i32)
                n4000 = Unbundle By Name(w6254) -> ("Y"=w6258:dbl[])
                n4001 = Subtract(x=w6252, y="N pts to average") -> (x-y=w6187:i32)
                n4002 = Multiply(x="N pts to average", y=u16 2) -> (x*y=w6230:u16)
                n4003 = Subtract(x=w6252, y=w6230) -> (x-y=w6188:i32)
                n4004 = feedback #36(w6258) -> (w6257:dbl[])
                n4005 = Build Array (concatenate)(w6257, w6258) -> (w6256:dbl[])
                n4006 = Select(t=w6258, s=w6179, f=w6256) -> (s? t:f=w6255:dbl[])
                "Trap Delta Graph" <- w6255
                n4007 = feedback-in #36(w6255) -> ()
                n4008 = Array Subset(array=w6234, index=w6187, length="N pts to average") -> (w6251:dbl[])
                n4009 = Array Subset(array=w6234, index=w6188, length="N pts to average") -> (w6250:dbl[])
                n4010 = Array Subset(array=w6229, index=w6187, length="N pts to average") -> (w6232:dbl[])
                n4011 = Array Subset(array=w6229, index=w6188, length="N pts to average") -> (w6231:dbl[])
                n4012 = Array Subset(array=w6190, index=w6187, length="N pts to average") -> (w6199:dbl[])
                n4013 = Array Subset(array=w6190, index=w6188, length="N pts to average") -> (w6198:dbl[])
                n4014 = Index Array(array=w6212, index=0) -> (element=w6210:waveform(dbl))
                n4015 = call-poly <vilib>:"Mean.vi"("X"=w6251) -> ("mean"=w6249:dbl)  [unwired: 1 out]
                n4016 = call-poly <vilib>:"Mean.vi"("X"=w6232) -> ("mean"=w6228:dbl)  [unwired: 1 out]
                n4017 = call-poly <vilib>:"Mean.vi"("X"=w6250) -> ("mean"=w6248:dbl)  [unwired: 1 out]
                n4018 = call-poly <vilib>:"Mean.vi"("X"=w6231) -> ("mean"=w6227:dbl)  [unwired: 1 out]
                n4019 = call-poly <vilib>:"Mean.vi"("X"=w6199) -> ("mean"=w6197:dbl)  [unwired: 1 out]
                n4020 = call-poly <vilib>:"Mean.vi"("X"=w6198) -> ("mean"=w6196:dbl)  [unwired: 1 out]
                n4021 = Unbundle By Name(w6210) -> ("Y"=w6208:dbl[])
                n4022 = Subtract(x=w6228, y=w6227) -> (x-y=w6219:dbl)
                "Delta Fl. 2" <- w6219
                n4023 = Subtract(x=w6197, y=w6196) -> (x-y=w6191:dbl)
                "Delta Fl. 3" <- w6191
                n4024 = Subtract(x=w6249, y=w6248) -> (x-y=w6246:dbl)
                "Delta Fl. 1" <- w6246
                n4025 = feedback #37(w6208) -> (w6207:dbl[])
                n4026 = Build Array (concatenate)(w6207, w6208) -> (w6209:dbl[])
                n4027 = Initialize Array(w6246, 1 ("dimension size")) -> (w6243:dbl[])
                n4028 = Initialize Array(w6219, 1 ("dimension size")) -> (w6224:dbl[])
                n4029 = Initialize Array(w6191, 1 ("dimension size")) -> (w6193:dbl[])
                n4030 = Select(t=w6208, s=w6179, f=w6209) -> (s? t:f=w6206:dbl[])
                "Saved trap pos" <- w6206
                n4031 = feedback-in #37(w6206) -> ()
                n4032 = feedback #38(w6243) -> (w6244:dbl[])
                n4033 = Build Array (concatenate)(w6244, w6243) -> (w6242:dbl[])
                n4034 = feedback #39(w6224) -> (w6225:dbl[])
                n4035 = feedback #40(w6193) -> (w6194:dbl[])
                n4036 = Build Array (concatenate)(w6225, w6224) -> (w6223:dbl[])
                n4037 = Build Array (concatenate)(w6194, w6193) -> (w6192:dbl[])
                n4038 = Select(t=w6243, s=w6179, f=w6242) -> (s? t:f=w6222:dbl[])
                n4039 = feedback-in #38(w6222) -> ()
                n4040 = Select(t=w6224, s=w6179, f=w6223) -> (s? t:f=w6221:dbl[])
                n4041 = feedback-in #39(w6221) -> ()
                n4042 = Select(t=w6193, s=w6179, f=w6192) -> (s? t:f=w6186:dbl[])
                n4043 = feedback-in #40(w6186) -> ()
                n4044 = Build Array(w6222, w6221, w6186) -> (→"Save APD Deriv":dbl[][])
                n4045 = Index Array(array=w6178, index=15) -> (element=w6184:waveform(dbl))
                n4046 = Unbundle By Name(w6184) -> ("Y"=w6182:dbl[])
                n4047 = feedback #41(w6182) -> (w6181:dbl[])
                n4048 = Build Array (concatenate)(w6181, w6182) -> (w6183:dbl[])
                n4049 = Select(t=w6182, s=w6179, f=w6183) -> (s? t:f=w6180:dbl[])
                "Amp current" <- w6180
                n4050 = feedback-in #41(w6180) -> ()
              }
            }
            "Progress" <- w6155
            "Progress 2" <- w6155
          }
        }
      }
    }
    n4051 = local read "wait to reset values"() -> (w4883:bool)
    n4052 = Not(x=w4881) -> (.not. x?=w4884:bool)
    n4053 = And(x=w4884, y=w4883) -> (x .and. y?=w4885:bool)
    n4054 = case "Part of MCL raster scanning: returns to initial positions after scan done" shown="True" w4885 {
      tunnel: w4567 -> [w5596 w5603]
      tunnel: [w5596 w5602] -> w4887
      tunnel: w4763 -> [w5595 w5601]
      tunnel: [w5595 w5600] -> w4882
      frame False {
      }
      frame True {
        w5611 = 10.0 ("y")
        w5610 = 32767.0 ("y")
        # "to return scan values\nafter a synchronous \nAOM scan"
        n4055 = local read "AO2"() -> (w5604:dbl)
        n4056 = local read "AO1"() -> (w5605:dbl)
        n4057 = local write "wait to reset values"(FALSE ("wait to reset values")) -> ()
        n4058 = Multiply(x=w5605, y=w5610) -> (x*y=w5607:dbl)
        n4059 = Multiply(x=w5604, y=w5610) -> (x*y=w5609:dbl)
        n4060 = Divide(x=w5607, y=w5611) -> (x/y=w5606:dbl)
        n4061 = Divide(x=w5609, y=w5611) -> (x/y=w5608:dbl)
        n4062 = To Word Integer(number=w5606) -> (16bit integer=w5612:i16)
        n4063 = To Word Integer(number=w5608) -> (16bit integer=w5613:i16)
        n4064 = local read "Total Counts (ticks)"() -> (w5597:u16)
        n4065 = local read "Scan Range (V)\n(of steps)"() -> (w5598:dbl)
        n4066 = xnode "Read/Write Control"("FPGA VI Reference In"=w5603, "error in"=w5601, "AO1 (Y)"=w5612, "AO2 (X)"=w5613, "MCL count"=w5597) -> ("FPGA VI Reference Out"=w5602:T40, "error out"=w5600:errorcluster)
        n4067 = property on="Scan Range (V)\n(of steps)" class="DigNum (strict)"("Val(Sgnl)"=w5598) -> ()  [unwired: 2 in, 2 out]
      }
    }
    n4068 = case shown="True" "Sound ON" {
      tunnel: [w5096 w5141] -> w4729
      tunnel: w4728 -> [w5096 w5140]
      tunnel: w4726 -> [_ _]
      tunnel: w4624 -> [_ w5099]
      tunnel: w4725 -> [_ _]
      tunnel: w4724 -> [_ w5110]
      tunnel: w4723 -> [_ w5120]
      frame False {
      }
      frame True {
        n4069 = Index Array(array=w5099, index="Data channel to sound") -> (element=w5098:waveform(dbl))
        "Waveform Graph 2" <- w5098
        n4070 = Unbundle By Name(w5098) -> ("dt"=w5124:dbl, "Y"=w5122:dbl[])
        n4071 = Array Size(array=w5122) -> (size(s)=w5123:i32)
        "N data samples" <- w5123
        n4072 = for "Data time base" {
          N: w5123 -> [_]
          tunnel: [w5145] -> w5125 mode=indexing
          i -> [w5145]
        }
        n4073 = Multiply(x=w5124, y=w5125) -> (x*y=w5121:dbl[])
        n4074 = Compound Arithmetic op=MULTIPLY(6.283185307179586, "Carrier Frequency (Hz)", w5120) -> (w5137:dbl[])
        n4075 = call <vilib>:"Interpolate 1D.vi"("X is monotonic"=TRUE, "xi"=w5120, "X"=w5121, "Y"=w5122) -> ("yi"=w5118:dbl[])  [unwired: 5 in, 2 out]
        n4076 = Sine(x=w5137) -> (sin(x)=w5126:dbl[])
        n4077 = Add(x=w5118, y="Offset") -> (x+y=w5116:dbl[])
        n4078 = Multiply(x=w5116, y="mult x") -> (x*y=w5114:dbl[])
        n4079 = Add(x="Offset 2", y=w5114) -> (x+y=w5109:dbl[])
        n4080 = Compound Arithmetic op=MULTIPLY(6.283185307179586, "Carrier Frequency (Hz)", w5110, w5109) -> (w5101:dbl[])
        n4081 = for "Cumulative sum" {
          tunnel: [w5144] -> w5107 mode=indexing
          shift-right: [w5144] -> w5104
          shift-left: 0.0 -> [w5143]
          tunnel: w5101 -> [w5142] mode=indexing
          n4082 = Add(x=w5142, y=w5143) -> (x+y=w5144:dbl)
        }
        n4083 = feedback #42(0.0) -> (w5103:dbl)
        n4084 = Add(x=w5107, y=w5103) -> (x+y=w5106:dbl[])
        n4085 = Add(x=w5104, y=w5103) -> (x+y=w5102:dbl)
        n4086 = feedback-in #42(w5102) -> ()
        n4087 = Sine(x=w5106) -> (sin(x)=w5100:dbl[])
        n4088 = Select(t=w5126, s="tone or data", f=w5100) -> (s? t:f=w5132:dbl[])
        n4089 = Multiply(x=w5132, y="Volume") -> (x*y=w5130:dbl[])
        n4090 = Initialize Array(0.0 ("element"), "N initial buffer elements") -> (w5133:dbl[])
        n4091 = Multiply(x="N initial buffer elements", y=w5110) -> (x*y=→"Initial buffer time (s)":dbl)
        n4092 = Build Array (concatenate)(w5133, w5130) -> (w5135:dbl[])
        n4093 = First Call?() -> (First Call?: T/F=w5136:bool)
        n4094 = Select(t=w5135, s=w5136, f=w5130) -> (s? t:f=w5129:dbl[])
        n4095 = call-poly <vilib>:"Sound Output Write.vi"("data"=w5129, "task ID"=w5140) -> ("task ID out"=w5141:T60)  [unwired: 8 in, 1 out]
      }
    }
    n4096 = node-c288() -> ()  [unwired: 2 out]
  }
  n4097 = disable-structure shown="Disabled" {
    disable-tunnel: w21 -> [w6323 _]
    frame Disabled {
      n4098 = call <vilib>:"Sound Output Clear.vi"("task ID"=w6323) -> ()  [unwired: 10 in, 1 out]
    }
    frame Enabled {
    }
  }
  n4099 = node-c288(w59) -> ()  [unwired: 1 out]
  n4100 = node-c288(w67) -> ()  [unwired: 1 out]
  n4101 = flat-sequence {
    tunnel: w74 -> [w6327]
    tunnel: w75 -> [w6328]
    tunnel: [w6326] -> w73
    tunnel: [w6325] -> w72
    tunnel: w71 -> [_]
    tunnel: w69 -> [_]
    tunnel: w65 -> [_]
    tunnel: w73 -> [w6329]
    tunnel: w72 -> [w6330]
    frame #0 {
      w6324 = FALSE ("AI to FIFO")
      n4102 = xnode "Read/Write Control"("FPGA VI Reference In"=w6328, "error in"=w6327, "AI to FIFO"=w6324, "APD to FIFO"=w6324) -> ("FPGA VI Reference Out"=w6326:T40, "error out"=w6325:errorcluster)
    }
    frame #1 {
      n4103 = xnode "Close FPGA VI Reference"("FPGA VI Reference In"=w6329, "error in"=w6330) -> ("error out"=→"error out":errorcluster)
    }
  }
